vi "UHR-Fleezers Control (host) - 12.7c.vi"() -> ()   [LabVIEW 2012] (continued)
          tunnel: w2948 -> [w2975]
          tunnel: w2947 -> [w2974]
          frame #0 {
            n2017 = call "Read Stage Position.vi"("error in"=w2965, "VISA resource name in"=w2957) -> ("Current Position"=w2955:cluster{dbl, dbl, dbl}, "error out"=w2958:errorcluster, "VISA resource name out"=w2956:refnum<visa-resource-name>)  [unwired: 1 out]
            "Current Position" <- w2955
            n2018 = local write "Stage Control Serial Error"(w2958) -> ()
            n2019 = Unbundle(w2955) -> (w2962:dbl, w2964:dbl, w2960:dbl)
            n2020 = Add(x=w2964, y="Y change (mm)") -> (x+y=w2961:dbl)
            n2021 = Bundle(w2962, w2961, w2960) -> (w2959:cluster{dbl, dbl, dbl})  [unwired: 1 in]
          }
          frame #1 {
            # "move to new position and start saving"
            n2022 = local write "Stage Moving"(TRUE ("Stage Moving")) -> ()
            n2023 = local write "Start Saving"(TRUE ("Start Saving")) -> ()
            n2024 = call "Set Stage Position.vi"("Position"=w2972, "error in"=w2971, "VISA resource name in"=w2970) -> ("error out"=w2968:errorcluster, "VISA resource name out"=w2969:refnum<visa-resource-name>)  [unwired: 1 out]
          }
          frame #2 {
            # "go back to start"
            n2025 = call "Set Stage Position.vi"("Position"=w2974, "error in"=w2975, "VISA resource name in"=w2976) -> ()  [unwired: 3 out]
          }
          frame #3 {
            # "stop saving"
            n2026 = local write "Stop Saving"(TRUE ("Stop Saving")) -> ()
            n2027 = local write "Stage Moving"(FALSE ("Stage Moving")) -> ()
          }
        }
      }
      event "Move to Position 1", "Move to Position 2", "Move to Position 3", "Move to Position 4", "Move to Position 5", "Lower Ch. Cap.": Value Change {
        n2028 = event-data() -> ()  [unwired: 1 in, 5 out]
        n2029 = Or(x="Move to Position 5", y="Lower Ch. Cap.") -> (x .or. y?=w2982:bool)
        n2030 = Build Array("Move to Position 1", "Move to Position 2", "Move to Position 3", "Move to Position 4", w2982) -> (w2985:bool[])
        n2031 = Boolean Array To Number(Boolean array=w2985) -> (number=w2984:u32)
        n2032 = Logarithm Base 2(1:w2984) -> (0:w2983:dbl)
        n2033 = flat-sequence {
          tunnel: w2983 -> [w2994]
          tunnel: w2980 -> [w2992]
          tunnel: w2979 -> [w2991]
          frame #0 {
            n2034 = local read "Saved Stage Positions"() -> (w3002:dbl[][])
            n2035 = Array Subset(array=w3002, index (row)=w2994, length (row)=1 ("length"), index (col)=1 ("index"), length (col)=3 ("length")) -> (w2999:dbl[][])
            n2036 = Reshape Array(w2999, 3 ("dimension size")) -> (w2997:dbl[])
            n2037 = Array To Cluster(array=w2997) -> (cluster=w2996:cluster{"[0]":dbl, "[1]":dbl, "[2]":dbl})
            n2038 = call "Set Stage Position.vi"("Position"=w2996, "error in"=w2991, "VISA resource name in"=w2992) -> ("error out"=w2995:errorcluster)  [unwired: 2 out]
            n2039 = local write "Stage Moving"(TRUE ("Stage Moving")) -> ()
            n2040 = local write "Stage Control Serial Error"(w2995) -> ()
          }
          frame #1 {
            n2041 = local write "Stage Moving"(FALSE ("Stage Moving")) -> ()
            n2042 = call <vilib>:"Beep.vi"() -> ()  [unwired: 3 in, 9 out]
          }
        }
      }
      event "Got ADig bead": Value Change {
        n2043 = event-data() -> ()  [unwired: 1 in, 5 out]
        n2044 = flat-sequence {
          frame #0 {
            n2045 = local read "Cap 1 Samp Flow ON"() -> (w3006:bool)
            n2046 = case shown="True" w3006 {
              frame False {
              }
              frame True {
                n2047 = property on="Sample Channel\nFlow" class="Bool (strict)"("Val(Sgnl)"=TRUE ("Value (Signaling)")) -> ()  [unwired: 2 in, 2 out]
              }
            }
          }
          frame #1 {
            n2048 = property on="Inject Pump 3" class="Bool (strict)"("Val(Sgnl)"=FALSE ("Value (Signaling)")) -> ()  [unwired: 2 in, 2 out]
          }
          frame #2 {
            n2049 = property on="Move Cap. 1 (DNA Bottom)" class="Bool (strict)"("Val(Sgnl)"=TRUE ("Value (Signaling)")) -> ()  [unwired: 2 in, 2 out]
          }
        }
      }
      event "Force FB Data\nScript": Value Change {
        n2050 = event-data() -> ()  [unwired: 1 in, 5 out]
        n2051 = flat-sequence {
          tunnel: w3015 -> [w3019]
          tunnel: w3016 -> [w3020]
          tunnel: [w3020] -> w3011
          tunnel: [w3019] -> w3010
          tunnel: w3011 -> [w3023]
          tunnel: w3010 -> [w3022]
          tunnel: ["Trap Trig Fl."] -> w3012
          tunnel: [w3048] -> w3013
          tunnel: w3012 -> [w3048]
          tunnel: [w3052] -> w3014
          tunnel: w3013 -> [w3052]
          tunnel: w3014 -> [w3054]
          frame #0 {
            n2052 = property on="Trap Delta (MHz)" class="DigNum (strict)"("Val(Sgnl)"="Trap Delta Before Moving") -> ()  [unwired: 2 in, 2 out]
          }
          frame #1 {
            n2053 = local read "Saved Stage Positions"() -> (w3025:dbl[][])
            n2054 = local write "FB Trap Pos Offset"(0.0 ("FB Trap Pos Offset")) -> ()
            n2055 = property on="Trap Pos. FB Offset Factor" class="DigNum (strict)"("Val(Sgnl)"=i64 0 ("Value (Signaling)")) -> ()  [unwired: 2 in, 2 out]
            n2056 = local write "Stage Moving"(TRUE ("Stage Moving")) -> ()
            n2057 = call "move to saved stage position.vi"("error in"=w3022, "Stage VISA resource name in"=w3023, "Position"="Stage Position To Establish FB", "Saved Stage Positions"=w3025) -> ("error out"=w3021:errorcluster)  [unwired: 1 out]
            n2058 = local write "Stage Control Serial Error"(w3021) -> ()
          }
          frame #2 {
            n2059 = call <vilib>:"Beep.vi"() -> ()  [unwired: 3 in, 9 out]
            n2060 = Multiply(x="Wait (s)", y=u32 1000 ("milliseconds to wait")) -> (x*y=w3032:u32)
            n2061 = property on="Trap Delta (MHz)" class="DigNum (strict)"("Val(Sgnl)"="Starting \nTrap Delta (MHz)") -> ()  [unwired: 2 in, 2 out]
            n2062 = local write "Stage Moving"(FALSE ("Stage Moving")) -> ()
            n2063 = Wait (ms)(milliseconds to wait=w3032) -> ()  [unwired: 1 out]
            n2064 = property on="Tab Control 2" class="TabCtl (strict)"("Val(Sgnl)"=T6."Feedback on Trap Position" ("Value (Signaling)")) -> ()  [unwired: 2 in, 2 out]
            n2065 = property on="Tab Control" class="TabCtl (strict)"("Val(Sgnl)"=T34."Trap Control (RF)" ("Value (Signaling)")) -> ()  [unwired: 2 in, 2 out]
          }
          frame #3 {
            n2066 = property on="Set Reading to\nSetpoint" class="Bool (strict)"("Val(Sgnl)"=TRUE ("Value (Signaling)")) -> ()  [unwired: 2 in, 2 out]
            n2067 = Wait (ms)(milliseconds to wait=u32 500) -> ()  [unwired: 1 out]
          }
          frame #4 {
            n2068 = property on="Trap Pos. FB ON" class="Bool (strict)"("Val(Sgnl)"=TRUE ("Value (Signaling)")) -> ()  [unwired: 2 in, 2 out]
            n2069 = Wait (ms)(milliseconds to wait=u32 250) -> ()  [unwired: 1 out]
          }
          frame #5 {
            n2070 = case shown="False" "Trap Trig Fl." {
              frame False {
                n2071 = case shown="True" "Green ON after FB ON?" {
                  selector: "Green ON after FB ON?" -> [_ w3047]
                  frame False {
                  }
                  frame True {
                    n2072 = property on="Green Laser ON" class="Bool (strict)"("Val(Sgnl)"=w3047) -> ()  [unwired: 2 in, 2 out]
                  }
                }
              }
              frame True {
              }
            }
            n2073 = case shown="True" "Remove Action Offset" {
              tunnel: TRUE ("Value (Signaling)") -> [w3044 w3045]
              frame False {
                n2074 = property on="Remove Unwinding Offset" class="Bool (strict)"("Val(Sgnl)"=w3044) -> ()  [unwired: 2 in, 2 out]
              }
              frame True {
                n2075 = property on="Remove Action Offset" class="Bool (strict)"("Val(Sgnl)"=w3045) -> ()  [unwired: 2 in, 2 out]
              }
            }
            n2076 = Wait (ms)(milliseconds to wait=u32 250) -> ()  [unwired: 1 out]
          }
          frame #6 {
            n2077 = property on="Start Saving" class="Bool (strict)"("Val(Sgnl)"=TRUE ("Value (Signaling)")) -> ()  [unwired: 2 in, 2 out]
            n2078 = Wait (ms)(milliseconds to wait=u32 5000) -> ()  [unwired: 1 out]
          }
          frame #7 {
            w3051 = TRUE ("Value (Signaling)")
            n2079 = property on="Rem fb disp offset" class="Bool (strict)"("Val(Sgnl)"=w3051) -> ()  [unwired: 2 in, 2 out]
            n2080 = property on="Remove Offset" class="Bool (strict)"("Val(Sgnl)"=w3051) -> ()  [unwired: 2 in, 2 out]
            n2081 = Wait (ms)(milliseconds to wait=u32 100) -> ()  [unwired: 1 out]
          }
          frame #8 {
            n2082 = case shown="True" w3054 {
              frame False {
              }
              frame True {
                n2083 = local write "Trap Trig. Fl."(TRUE ("Value (Signaling)")) -> ()
              }
            }
          }
          frame #9 {
            n2084 = case shown="True" "Start dipping after?" {
              frame False {
              }
              frame True {
                n2085 = flat-sequence {
                  frame #0 {
                    n2086 = Multiply(x="Delay before dipping (s)", y=1000.0) -> (x*y=w3058:dbl)
                    n2087 = Wait (ms)(milliseconds to wait=w3058) -> ()  [unwired: 1 out]
                  }
                  frame #1 {
                    n2088 = property on="Dip for Protein" class="Bool (strict)"("Val(Sgnl)"=TRUE ("Value (Signaling)")) -> ()  [unwired: 2 in, 2 out]
                    n2089 = local write "Scripts"(T1."Dipping" ("Scripts")) -> ()
                  }
                }
              }
            }
          }
        }
      }
      event "Fixed Traps Data\nScript": Value Change {
        n2090 = event-data() -> ()  [unwired: 1 in, 5 out]
        n2091 = flat-sequence {
          frame #0 {
            n2092 = case shown="True" "Green ON" {
              frame False {
              }
              frame True {
                n2093 = property on="Green Laser ON" class="Bool (strict)"("Val(Sgnl)"=TRUE) -> ()  [unwired: 2 in, 2 out]
              }
            }
            n2094 = local write "Offset (nm)"(0.0 ("Offset (nm)")) -> ()
            n2095 = property on="Sample Channel\nFlow" class="Bool (strict)"("Val(Sgnl)"=FALSE ("Value (Signaling)")) -> ()  [unwired: 2 in, 2 out]
            n2096 = property on="Trap Delta (MHz)" class="DigNum (strict)"("Val(Sgnl)"="Fixed Traps Trap Delta (MHz)") -> ()  [unwired: 2 in, 2 out]
          }
          frame #1 {
            n2097 = Wait (ms)(milliseconds to wait=u32 1000) -> ()  [unwired: 1 out]
          }
          frame #2 {
            n2098 = local write "Start Saving"(TRUE ("Start Saving")) -> ()
          }
          frame #3 {
            n2099 = local read "Bead Sep. Int. Time (s)"() -> (w3069:dbl)
            n2100 = Multiply(x=w3069, y=1000.0) -> (x*y=w3071:dbl)
            n2101 = Wait (ms)(milliseconds to wait=w3071) -> ()  [unwired: 1 out]
          }
          frame #4 {
            n2102 = property on="Remove Offset" class="Bool (strict)"("Val(Sgnl)"=TRUE ("Value (Signaling)")) -> ()  [unwired: 2 in, 2 out]
          }
          frame #5 {
            n2103 = property on="Dip for Protein" class="Bool (strict)"("Val(Sgnl)"="Start dipping after?") -> ()  [unwired: 2 in, 2 out]
          }
        }
      }
      event "Got DNA bead": Value Change {
        n2104 = event-data() -> ()  [unwired: 1 in, 5 out]
        n2105 = flat-sequence {
          frame #0 {
            n2106 = local read "Daq spot flow on"() -> (w3076:bool)
            n2107 = case shown="True" w3076 {
              frame False {
              }
              frame True {
                n2108 = property on="Sample Channel\nFlow" class="Bool (strict)"("Val(Sgnl)"=TRUE ("Value (Signaling)")) -> ()  [unwired: 2 in, 2 out]
              }
            }
            n2109 = property on="Got DNA bead" class="Bool"("Key Focus"=FALSE) -> ()  [unwired: 2 in, 2 out]
          }
          frame #1 {
            n2110 = property on="Inject Pump 1" class="Bool (strict)"("Val(Sgnl)"=FALSE ("Value (Signaling)")) -> ()  [unwired: 2 in, 2 out]
          }
          frame #2 {
            n2111 = property on="Cal/Data Acq. Spot" class="Bool (strict)"("Val(Sgnl)"=TRUE ("Value (Signaling)")) -> ()  [unwired: 2 in, 2 out]
          }
        }
      }
      event "Take Stepping Data": Value Change {
        n2112 = event-data() -> ()  [unwired: 1 in, 5 out]
        n2113 = local read "Save ave N"() -> (w3088:dbl)
        n2114 = flat-sequence {
          tunnel: w3088 -> [w3090]
          tunnel: [w3090] -> w3083
          tunnel: [w3092] -> w3084
          tunnel: w3083 -> [w3092]
          tunnel: [w3094] -> w3085
          tunnel: w3084 -> [w3094]
          tunnel: [w3097] -> w3086
          tunnel: w3085 -> [w3097]
          tunnel: [w3099] -> w3087
          tunnel: w3086 -> [w3099]
          tunnel: [w3101] -> w3081
          tunnel: w3087 -> [w3101]
          tunnel: w3081 -> [w3104]
          tunnel: [w3104] -> w3080
          tunnel: w3080 -> [w3105]
          tunnel: [w3105] -> w3082
          tunnel: w3082 -> [w3111]
          frame #0 {
            n2115 = property on="Save ave N" class="DigNum (strict)"("Val(Sgnl)"="Save ave factor") -> ()  [unwired: 2 in, 2 out]
          }
          frame #1 {
            n2116 = Wait (ms)(milliseconds to wait=u32 100) -> ()  [unwired: 1 out]
          }
          frame #2 {
            n2117 = local read "Offset 2 Start (MHz)"() -> (w3096:dbl)
            n2118 = property on="Saved AOD Raster Scan Parameter Sets" class="Arr (strict)"("Index Values"=u32[] [2]) -> ()  [unwired: 2 in, 2 out]
            n2119 = property on="Trap Delta (MHz)" class="DigNum (strict)"("Val(Sgnl)"=w3096) -> ()  [unwired: 2 in, 2 out]
          }
          frame #3 {
            n2120 = property on="Load parameters" class="Bool (strict)"("Val(Sgnl)"=TRUE ("Value (Signaling)")) -> ()  [unwired: 2 in, 2 out]
          }
          frame #4 {
            n2121 = Wait (ms)(milliseconds to wait=u32 100) -> ()  [unwired: 1 out]
          }
          frame #5 {
            n2122 = property on="Trap Raster Scan" class="Bool (strict)"("Val(Sgnl)"=TRUE ("Value (Signaling)")) -> ()  [unwired: 2 in, 2 out]
          }
          frame #6 {
            n2123 = Wait (ms)(milliseconds to wait=u32 1000) -> ()  [unwired: 1 out]
          }
          frame #7 {
            n2124 = while {
              stop <- w3108 stop-if-true
              n2125 = local read "Raster Scanning..."() -> (w3110:bool)
              n2126 = local read "Saving..."() -> (w3109:bool)
              n2127 = Not(x=w3109) -> (.not. x?=w3106:bool)
              n2128 = Not(x=w3110) -> (.not. x?=w3107:bool)
              n2129 = And(x=w3107, y=w3106) -> (x .and. y?=w3108:bool)
            }
          }
          frame #8 {
            n2130 = property on="Save ave N" class="DigNum (strict)"("Val(Sgnl)"=w3111) -> ()  [unwired: 2 in, 2 out]
          }
        }
      }
      event "Step Size (nm)": Value Change {
        n2131 = event-data() -> ()  [unwired: 1 in, 5 out]
        n2132 = flat-sequence {
          frame #0 {
            n2133 = property on="Saved AOD Raster Scan Parameter Sets" class="Arr (strict)"("Index Values"=u32[] [1]) -> ()  [unwired: 2 in, 2 out]
          }
          frame #1 {
            n2134 = Multiply(x="N Steps", y="Step Size (nm)") -> (x*y=w3113:dbl)
            n2135 = property on="Scan Speed AOD (nm/s) 2" class="DigNum (strict)"("Value"="Step Size (nm)") -> ()  [unwired: 2 in, 2 out]
            n2136 = property on="Step Size AOD (nm) 2" class="DigNum (strict)"("Value"="Step Size (nm)") -> ()  [unwired: 2 in, 2 out]
            n2137 = property on="Scan Range AOD (nm) 2" class="DigNum (strict)"("Value"=w3113) -> ()  [unwired: 2 in, 2 out]
          }
        }
      }
      event "Take Detection Laser\nImage": Value Change {
        n2138 = event-data() -> ()  [unwired: 1 in, 5 out]
        n2139 = flat-sequence {
          tunnel: [w3141] -> w3131
          tunnel: [w3140] -> w3124
          tunnel: [w3139] -> w3116
          tunnel: [w3144] -> w3132
          tunnel: w3131 -> [w3144]
          tunnel: [w3143] -> w3125
          tunnel: w3124 -> [w3143]
          tunnel: [w3142] -> w3117
          tunnel: w3116 -> [w3142]
          tunnel: [w3148] -> w3133
          tunnel: w3132 -> [w3148]
          tunnel: [w3147] -> w3126
          tunnel: w3125 -> [w3147]
          tunnel: [w3146] -> w3118
          tunnel: w3117 -> [w3146]
          tunnel: [w3154] -> w3134
          tunnel: w3133 -> [w3154]
          tunnel: [w3153] -> w3127
          tunnel: w3126 -> [w3153]
          tunnel: [w3152] -> w3119
          tunnel: w3118 -> [w3152]
          tunnel: [w3158] -> w3135
          tunnel: w3134 -> [w3158]
          tunnel: [w3157] -> w3128
          tunnel: w3127 -> [w3157]
          tunnel: [w3156] -> w3120
          tunnel: w3119 -> [w3156]
          tunnel: [w3162] -> w3136
          tunnel: w3135 -> [w3162]
          tunnel: [w3161] -> w3129
          tunnel: w3128 -> [w3161]
          tunnel: [w3160] -> w3121
          tunnel: w3120 -> [w3160]
          tunnel: [w3166] -> w3137
          tunnel: w3136 -> [w3166]
          tunnel: [w3165] -> w3130
          tunnel: w3129 -> [w3165]
          tunnel: [w3164] -> w3122
          tunnel: w3121 -> [w3164]
          tunnel: w3137 -> [w3172]
          tunnel: w3130 -> [w3171]
          tunnel: [w3169] -> w3123
          tunnel: w3122 -> [w3169]
          tunnel: w3123 -> [w3173]
          frame #0 {
            n2140 = local read "Laser interlacing mode"() -> (w3140:enum32{"Laser ON", "Laser OFF", "Interlace"})
            n2141 = local read "Green FB On/Off"() -> (w3139:bool)
            n2142 = local read "Green Laser ON"() -> (w3141:bool)
          }
          frame #1 {
            n2143 = property on="Green FB On/Off" class="Bool (strict)"("Val(Sgnl)"=FALSE ("Value (Signaling)")) -> ()  [unwired: 2 in, 2 out]
          }
          frame #2 {
            n2144 = property on="Green Laser ON" class="Bool (strict)"("Val(Sgnl)"=TRUE ("Value (Signaling)")) -> ()  [unwired: 2 in, 2 out]
            n2145 = property on="Flip Green Filter" class="Bool (strict)"("Val(Sgnl)"=TRUE ("Value (Signaling)")) -> ()  [unwired: 2 in, 2 out]
            n2146 = property on="Laser interlacing mode" class="RadioBtnsControl (strict)"("Val(Sgnl)"=enum32{"Laser ON", "Laser OFF", "Interlace"}."Laser ON" ("Value (Signaling)")) -> ()  [unwired: 2 in, 2 out]
          }
          frame #3 {
            n2147 = Wait (ms)(milliseconds to wait=u32 500) -> ()  [unwired: 1 out]
          }
          frame #4 {
            n2148 = property on="Confocal Image" class="Bool (strict)"("Val(Sgnl)"=TRUE ("Value (Signaling)")) -> ()  [unwired: 2 in, 2 out]
          }
          frame #5 {
            n2149 = Wait (ms)(milliseconds to wait=u32 2000) -> ()  [unwired: 1 out]
          }
          frame #6 {
            n2150 = while {
              stop <- w3167 stop-if-true
              n2151 = local read "Saving..."() -> (w3168:bool)
              n2152 = Not(x=w3168) -> (.not. x?=w3167:bool)
            }
          }
          frame #7 {
            n2153 = property on="Flip Green Filter" class="Bool (strict)"("Val(Sgnl)"=TRUE ("Value (Signaling)")) -> ()  [unwired: 2 in, 2 out]
            n2154 = property on="Green Laser ON" class="Bool (strict)"("Val(Sgnl)"=w3172) -> ()  [unwired: 2 in, 2 out]
            n2155 = property on="Laser interlacing mode" class="RadioBtnsControl (strict)"("Val(Sgnl)"=w3171) -> ()  [unwired: 2 in, 2 out]
          }
          frame #8 {
            n2156 = property on="Green FB On/Off" class="Bool (strict)"("Val(Sgnl)"=w3173) -> ()  [unwired: 2 in, 2 out]
          }
        }
      }
      event "Move in a Circle": Value Change {
        w3184 = dbl[] []
        # "converting distance (d) to angle (a)\na=arcsin(d/2r)"
        # "radius"
        # "radius"
        # "T1 Y"
        # "T1 X"
        n2157 = event-data() -> ()  [unwired: 1 in, 5 out]
        n2158 = local read "BD 1 Frequency 1 (MHz)"() -> (w3181:dbl)
        n2159 = local read "BD 2 Frequency 1 (MHz)"() -> (w3180:dbl)
        n2160 = local read "BD 1 Frequency 2 (MHz)"() -> (w3179:dbl)
        n2161 = local read "BD 2 Frequency 2 (MHz)"() -> (w3178:dbl)
        n2162 = Subtract(x=w3180, y="Center Y Frequency (MHz)") -> (x-y=w3186:dbl)
        n2163 = Absolute Value(x=w3186) -> (abs(x)=w3176:dbl)
        n2164 = flat-sequence {
          tunnel: w3176 -> [w3189]
          tunnel: [w3189] -> w3175
          frame #0 {
            n2165 = local write "Radius (MHz)"(w3189) -> ()
          }
        }
        n2166 = node-c288("Time step (ms)") -> (w3188:T23)  [unwired: 3 in]
        n2167 = timed-loop {
          timing: w3188 -> [_]
          timing-out: [_] -> w3187
          tunnel: w3181 -> [w3246]
          tunnel: w3180 -> [_]
          tunnel: w3179 -> [w3250]
          tunnel: w3178 -> [_]
          tunnel: "Center Y Frequency (MHz)" -> [w3227]
          shift-right: [w3237] -> _
          shift-left: w3184 -> [w3239]
          shift-right: [w3236] -> _
          shift-left: w3184 -> [w3238]
          shift-right: [w3234] -> _
          shift-left: w3184 -> [w3233]
          shift-right: [w3232] -> _
          shift-left: w3184 -> [w3231]
          tunnel: "Move in a Circle" -> [_]
          tunnel: ["Back to start on finish?"] -> w3177
          tunnel: w3175 -> [_]
          tunnel: w3174 -> [w3204]
          i -> [w3226]
          stop <- w3244 stop-if-true
          # "Trap 2"
          # "Trap 1"
          # "ignore if N = 0"
          # "r"
          # "r"
          # "r"
          # "r"
          # "\"omega*t\""
          # "Trap 2"
          # "Trap separation (radians)"
          # "Trap 1"
          # "Offset (starts\n at bottom of\n the circle)"
          # "\"t\""
          # "omega"
          n2168 = node-c288() -> (w3259:i64)  [unwired: 1 in]
          n2169 = Divide(x=w3259, y=1000) -> (x/y=w3258:dbl)
          n2170 = Divide(x="2D Motion Trap Separation (MHz)", y="Radius (MHz)") -> (x/y=w3214:dbl)
          n2171 = Multiply(x=w3258, y=w3226) -> (x*y=w3218:dbl)
          n2172 = Inverse Sine(1:w3214) -> ()  [unwired: 1 out]
          n2173 = Multiply(x=w3218, y=-1.0) -> (x*y=w3219:dbl)
          n2174 = Multiply(x=6.283185307179586, y="2D Motion Frequency (Hz)") -> (x*y=w3229:dbl)
          n2175 = Select(t=w3218, s="Counterclockwise/Clockwise", f=w3219) -> (s? t:f=w3217:dbl)
          n2176 = Multiply(x=w3229, y=w3217) -> (x*y=w3240:dbl)
          n2177 = Divide(x="Trap 2 phase shift (deg)", y=6.283185307179586) -> (x/y=w3199:dbl)
          n2178 = Add(x=w3240, y=w3199) -> (x+y=w3211:dbl)
          n2179 = Add(x=w3240, y=1.5707963267948966) -> (x+y=w3256:dbl)
          n2180 = Add(x=w3211, y=1.5707963267948966) -> (x+y=w3241:dbl)
          n2181 = Cosine(x=w3256) -> (cos(x)=w3255:dbl)
          n2182 = Sine(x=w3256) -> (sin(x)=w3254:dbl)
          n2183 = Multiply(x=w3255, y="Radius (MHz)") -> (x*y=w3248:dbl)
          n2184 = Cosine(x=w3241) -> (cos(x)=w3253:dbl)
          n2185 = Sine(x=w3241) -> (sin(x)=w3252:dbl)
          n2186 = Multiply(x=w3254, y="Radius (MHz)") -> (x*y=w3247:dbl)
          n2187 = Multiply(x=w3253, y="Radius (MHz)") -> (x*y=w3251:dbl)
          n2188 = Multiply(x=w3252, y="Radius (MHz)") -> (x*y=w3249:dbl)
          n2189 = Add(x=w3248, y=w3246) -> (x+y=w3210:dbl)
          n2190 = Add(x=w3247, y=w3227) -> (x+y=w3208:dbl)
          n2191 = Greater Or Equal?(x=w3226, y="N steps then stop") -> (x >= y?=w3225:bool)
          n2192 = Add(x=w3251, y=w3250) -> (x+y=w3209:dbl)
          n2193 = Add(x=w3249, y=w3227) -> (x+y=w3207:dbl)
          n2194 = Not Equal To 0?(x="N steps then stop") -> (x != 0?=w3221:bool)
          n2195 = And(x=w3225, y=w3221) -> (x .and. y?=w3222:bool)
          n2196 = local read "Stop All"() -> (w3243:bool)
          n2197 = local write "BD 1 Frequency 1 (MHz)"(w3210) -> ()
          n2198 = local write "BD 2 Frequency 1 (MHz)"(w3208) -> ()
          n2199 = local write "BD 1 Frequency 2 (MHz)"(w3209) -> ()
          n2200 = local write "BD 2 Frequency 2 (MHz)"(w3207) -> ()
          n2201 = Compound Arithmetic op=OR(w3243, "Stop Moving", w3222) -> (w3244:bool)
          n2202 = local read "BD 1 Frequency 3 (MHz)"() -> (w3206:dbl)
          n2203 = local read "BD 2 Frequency 3 (MHz)"() -> (w3205:dbl)
          n2204 = local read "Y RF Frequency Limits (MHz)"() -> (w3202:T16)
          n2205 = local read "X RF Frequency Limits (MHz)"() -> (w3203:T16)
          n2206 = call "set RF board frequency - interlace.vi"("Board 2 Frequency Limits"=w3202, "Board 1 Frequency Limits"=w3203, "FPGA VI Reference In"=w3204, "Board 2 Frequency 3 (MHz)"=w3205, "Board 1 Frequency 3 (MHz)"=w3206, "Board 2 Frequency 2 (MHz)"=w3207, "Board 2 Frequency 1 (MHz)"=w3208, "Board 1 Frequency 2 (MHz)"=w3209, "Board 1 Frequency 1  (MHz)"=w3210) -> ()  [unwired: 1 in, 2 out]
          n2207 = Build Array (concatenate)(w3239, w3210) -> (w3237:dbl[])
          n2208 = Build Array (concatenate)(w3238, w3208) -> (w3236:dbl[])
          n2209 = Build Array (concatenate)(w3233, w3209) -> (w3234:dbl[])
          n2210 = Build Array (concatenate)(w3231, w3207) -> (w3232:dbl[])
          n2211 = Bundle(w3237, w3236) -> (→"Trap 1 trajectory":cluster{dbl[], dbl[]})  [unwired: 1 in]
          n2212 = Bundle(w3234, w3232) -> (→"Trap 2 trajectory":cluster{dbl[], dbl[]})  [unwired: 1 in]
          n2213 = node-c288() -> ()  [unwired: 1 in, 1 out]
        }
        n2214 = node-c288(w3187) -> ()  [unwired: 1 out]
        n2215 = case shown="True" w3177 {
          tunnel: w3181 -> [_ w3193]
          tunnel: w3180 -> [_ w3192]
          tunnel: w3179 -> [_ w3191]
          tunnel: w3178 -> [_ w3190]
          frame False {
          }
          frame True {
            n2216 = flat-sequence {
              tunnel: w3193 -> [w3197]
              tunnel: w3192 -> [w3196]
              tunnel: w3191 -> [w3195]
              tunnel: w3190 -> [w3194]
              frame #0 {
                n2217 = local write "BD 1 Frequency 1 (MHz)"(w3197) -> ()
                n2218 = local write "BD 2 Frequency 1 (MHz)"(w3196) -> ()
                n2219 = local write "BD 1 Frequency 2 (MHz)"(w3195) -> ()
                n2220 = local write "BD 2 Frequency 2 (MHz)"(w3194) -> ()
              }
              frame #1 {
                n2221 = property on="Update all trap values" class="Bool (strict)"("Val(Sgnl)"=TRUE ("Value (Signaling)")) -> ()  [unwired: 2 in, 2 out]
              }
            }
          }
        }
      }
      event "Stop All": Value Change {
        # "Stopping blue laser before shutting off program"
        n2222 = event-data() -> ()  [unwired: 1 in, 5 out]
        n2223 = local read "Delay (ms)"() -> (w3270:i32)
        n2224 = call "serial write macro.vi"("String"="l0", "Delay (ms)"=w3270, "VISA resource name"=w3273) -> ("read buffer"=w3268:string, "error out"=w3269:errorcluster, "VISA resource name out"=w3272:refnum<visa-resource-name>)
        n2225 = local write "read blue buffer"(w3268) -> ()
        n2226 = local write "Blue Error Out"(w3269) -> ()
        n2227 = VISA Close(VISA resource name=w3272) -> ()  [unwired: 1 in, 1 out]
        n2228 = local read "Stop All"() -> (w3274:bool)
      }
    }
    n2229 = node-c288() -> ()  [unwired: 1 in, 1 out]
  }
  n2230 = flat-sequence "Video" {
    tunnel: [w3284] -> w121
    tunnel: w121 -> [w3324]
    frame #0 {
      n2231 = while {
        stop <- w3276 continue-if-true
        n2232 = call "Close Video Capture.vi"() -> ("error code OUT"=w3278:i32)
        n2233 = Equal?(x=w3278, y=0) -> (x = y?=w3276:bool)
      }
      n2234 = local write "Stop All"(FALSE ("Stop All")) -> ()
    }
    frame #1 {
      n2235 = call "DMR_Init.vi"() -> ()  [unwired: 3 out]
    }
    frame #2 {
      w3279 = "DE245428202"  # MSU fleezers card #
      (unwired) "DE019116701"  # Illinois fleezers card #
      # "Setting the destination format to Mono8 makes sure that the image can be displayed in the intensity plot."
      n2236 = call "DMR_GetDevice.vi"("search string IN"=w3279) -> ("device handle OUT"=w3302:i32)  [unwired: 4 in, 2 out]
      n2237 = call "DMR_OpenDevice.vi"("device handle IN"=w3302) -> ("driver handle OUT"=w3285:i32)  [unwired: 4 out]
      n2238 = call "DMR_FindList.vi"("flags IN"=u32 0 ("flags"), "list name IN"="" ("String"), "list type IN"=T35."camera descriptions", "driver handle IN"=w3285) -> ("list handle OUT"=w3288:i32)  [unwired: 2 out]
      n2239 = call "DMR_FindList.vi"("flags IN"=u32 0 ("flags"), "list name IN"="Base", "list type IN"=T35."setting", "driver handle IN"=w3285) -> ("list handle OUT"=w3286:i32)  [unwired: 2 out]
      n2240 = call "OBJ_GetHandle.vi"("object name IN"="VideoStandard", "list handle IN"=w3288) -> ("object handle OUT"=w3282:i32)  [unwired: 3 out]
      n2241 = call "OBJ_GetHandle.vi"("object name IN"="PixelFormat", "list handle IN"=w3286) -> ("object handle OUT"=w3296:i32)  [unwired: 3 out]
      n2242 = call "OBJ_SetS.vi"("value index IN"=0, "value IN"="NTSC M", "object handle IN"=w3282) -> ()  [unwired: 2 out]
      n2243 = call "OBJ_SetS.vi"("value index IN"=0, "value IN"="Mono8" ("value"), "object handle IN"=w3296) -> ()  [unwired: 2 out]
      n2244 = call "OBJ_GetHandle.vi"("object name IN"="VideoChannel", "list handle IN"=w3286) -> ("object handle OUT"=w3292:i32)  [unwired: 3 out]
      n2245 = while {
        tunnel: [w3306] -> w3284
        tunnel: w3285 -> [w3303]
        stop <- w3304 continue-if-true
        n2246 = call "DMR_ImageRequestSingle.vi"("request control IN"=0, "driver handle IN"=w3303) -> ("error code OUT"=w3305:i32, "driver handle OUT"=w3306:i32)  [unwired: 2 out]
        n2247 = Equal To 0?(x=w3305) -> (x = 0?=w3304:bool)
      }
      n2248 = call "OBJ_SetI.vi"("value index IN"=0, "value IN"=3 ("Video channel"), "object handle IN"=w3292) -> ()  [unwired: 2 out]
    }
    frame #3 {
      w3312 = T18 0 items=["Grayscale (U8)", "Grayscale (I16)", "Grayscale (SGL)", "Complex (CSG)", "RGB (U32)", "HSL (U32)", "RGB (U64)"] ("Image Type")
      w3320 = T18 0 items=["Grayscale (U8)", "Grayscale (I16)", "Grayscale (SGL)", "Complex (CSG)", "RGB (U32)", "HSL (U32)", "RGB (U64)"] ("Image Type")
      n2249 = for "Create Greyscale map" {
        N: 256 -> [_]
        tunnel: [w3326] -> w3309 mode=indexing
        workers-P: _ -> [_]
        i -> [w3329]
        n2250 = To Unsigned Byte Integer(number=w3329) -> (unsigned 8bit integer=w3325:u8)
        n2251 = Join Numbers(hi=w3325, lo=w3325) -> ((hi.lo)=w3328:u16)
        n2252 = Join Numbers(hi=w3325, lo=w3325) -> ((hi.lo)=w3327:u16)
        n2253 = Join Numbers(hi=w3328, lo=w3327) -> ((hi.lo)=w3326:u32)
      }
      n2254 = call "IMAQ Create"("Image Name"="Scaled video", "Image Type"=w3312) -> ("New Image"=w3311:T2)  [unwired: 2 in, 2 out]
      n2255 = call "IMAQ Create"("Image Name"="Main video", "Image Type"=w3320) -> ("New Image"=w3321:T2)  [unwired: 2 in, 2 out]
      n2256 = node-c288(0 ("Processor")) -> (w3319:T23)  [unwired: 3 out]
      n2257 = Initialize Array(u32 0 ("Window Number (0...15)"), 480 ("dimension size"), 640 ("dimension size")) -> (w3314:u32[][])
      n2258 = timed-loop {
        tunnel: w3324 -> [w3346]
        tunnel: [w3345] -> w3323
        tunnel: w3321 -> [w3344]
        timing: w3319 -> [_]
        timing-out: [_] -> w3318
        tunnel: w3314 -> [w3333]
        tunnel: w3311 -> [w3331]
        tunnel: w3309 -> [w3330]
        stop <- w3332 stop-if-true
        # "This block performs the \nactual image capture."
        n2259 = node-c288() -> ()  [unwired: 2 out]
        n2260 = local read "Stop All"() -> (w3332:bool)
        n2261 = Reciprocal(x="Video Capture Rate (Hz)") -> (1/x=w3336:dbl)
        n2262 = Multiply(x=w3336, y=1000.0) -> (x*y=w3334:dbl)
        n2263 = call "DMR_ImageRequestWaitFor.vi"("queue number IN"=0, "timeout(ms) IN"=500, "driver handle IN"=w3346) -> ("error code OUT"=w3350:i32, "request number OUT"=w3347:i32, "driver handle OUT"=w3348:i32)
        n2264 = feedback #1(T36 refnum ("Avi Refnum")) -> (w3338:T36)
        n2265 = case shown="True" "New Video File" {
          tunnel: [T36 refnum ("Avi Refnum") w3367] -> w3340
          tunnel: [FALSE TRUE] -> w3341
          tunnel: w3338 -> [_ w3363]
          frame False {
          }
          frame True {
            n2266 = call "Create new save file.vi"("Ext"=".avi" ("string"), "Index In"="Video Index") -> ("Path Out"=w3359:path, "Index Out"=w3360:dbl)  [unwired: 1 in]
            "Path Out" <- w3359
            n2267 = Not Equal?(x=w3363, y=T36 refnum ("Avi Refnum")) -> (x != y?=w3364:bool)
            n2268 = Increment(x=w3360) -> (x+1=w3369:dbl)
            n2269 = case shown="True" w3364 {
              tunnel: w3363 -> [_ w3370]
              frame False {
              }
              frame True {
                n2270 = call "IMAQ AVI Close"("Avi Refnum"=w3370) -> ()  [unwired: 1 in, 10 out]
              }
            }
            n2271 = local write "Video Index"(w3369) -> ()
            n2272 = call "IMAQ AVI Create"("Frames Per Second"=u32 30, "AVI Path"=w3359) -> ("Avi Refnum"=w3367:T36)  [unwired: 5 in, 4 out]
          }
        }
        n2273 = Equal To 0?(x=w3350) -> (x = 0?=w3349:bool)
        n2274 = Select(t=w3340, s=w3341, f=w3338) -> (s? t:f=w3339:T36)
        n2275 = feedback-in #1(w3339) -> ()
        n2276 = case shown="True" w3349 {
          tunnel: w3348 -> [w3371 w3405]
          tunnel: w3347 -> [_ w3404]
          tunnel: [w3371 w3401] -> w3345
          tunnel: w3344 -> [_ w3386]
          tunnel: w3333 -> [_ w3390]
          tunnel: w3339 -> [_ w3388]
          tunnel: w3331 -> [_ w3383]
          tunnel: w3330 -> [_ w3382]
          frame False {
          }
          frame True {
            w3395 = u32 0 ("X-offset IN")
            n2277 = call "DMR_GetImageRequestBufferData.vi"("driver handle IN"=w3405, "request number IN"=w3404) -> ("width OUT"=w3394:i32, "height OUT"=w3393:i32, "driver handle OUT"=w3400:i32, "request number OUT"=w3399:i32, "bytes per pixel OUT"=w3396:i32)  [unwired: 13 out]
            n2278 = call "DMR_GetImageRequestBufferImageData.vi"("driver handle IN"=w3400, "request number IN"=w3399, "bytes per pixel IN"=w3396, "X-offset IN"=w3395, "Y-offset IN"=w3395, "height IN"=w3393, "width IN"=w3394) -> ("driver handle OUT"=w3398:u32, "request number OUT"=w3397:u32, "image OUT"=w3375:u32[][])  [unwired: 10 out]
            n2279 = Transpose 2D Array(2D array=w3375) -> (transposed array=w3381:u32[][])
            n2280 = Select(t=w3381, s="Flip Y (or X)", f=w3375) -> (s? t:f=w3380:u32[][])
            n2281 = call "DMR_ImageRequestUnlock.vi"("request number IN"=w3397, "driver handle IN"=w3398) -> ("driver handle OUT"=w3403:i32)  [unwired: 1 in, 2 out]
            n2282 = for {
              tunnel: w3380 -> [w3440] mode=indexing
              tunnel: [w3439] -> w3378 mode=indexing
              n2283 = Reverse 1D Array(array=w3440) -> (reversed array=w3439:u32[])
            }
            n2284 = call "DMR_ImageRequestSingle.vi"("request control IN"=0, "driver handle IN"=w3403) -> ("driver handle OUT"=w3401:i32)  [unwired: 3 out]
            n2285 = Transpose 2D Array(2D array=w3378) -> (transposed array=w3379:u32[][])
            n2286 = Select(t=w3379, s="Flip Y (or X)", f=w3378) -> (s? t:f=w3376:u32[][])
            n2287 = Select(t=w3376, s="Flip Image", f=w3375) -> (s? t:f=w3373:u32[][])
            n2288 = case shown="True" "Averaging" {
              tunnel: w3373 -> [w3443 w3448]
              tunnel: [w3443 w3447] -> w3387
              tunnel: w3390 -> [_ w3445]
              frame False {
              }
              frame True {
                (unwired) 1
                w3453 = 1
                n2289 = feedback #2(w3445) -> (w3444:u32[][])
                n2290 = Add(x=w3448, y=w3444) -> (x+y=w3449:u32[][])
                n2291 = Select(t=w3445, s="Reset Averaging", f=w3449) -> (s? t:f=w3451:u32[][])
                n2292 = feedback-in #2(w3451) -> ()
                n2293 = feedback #3(w3453) -> (w3446:i32)
                n2294 = Divide(x=w3449, y=w3446) -> (x/y=w3450:dbl[][])
                n2295 = Increment(x=w3446) -> (x+1=w3454:i32)
                n2296 = To Unsigned Long Integer(number=w3450) -> (unsigned 32bit integer=w3447:u32[][])
                n2297 = Select(t=w3453, s="Reset Averaging", f=w3454) -> (s? t:f=w3452:i32)
                n2298 = feedback-in #3(w3452) -> ()
              }
            }
            n2299 = case shown="True" "Zoom video window" {
              tunnel: w3387 -> [_ w3419]
              tunnel: w3383 -> [_ w3418]
              frame False {
              }
              frame True {
                n2300 = To Double Precision Float(number=w3419) -> (double precision float=w3416:dbl[][])
                n2301 = In Range and Coerce(upper limit="Intensity Upper", x=w3416, lower limit="Intensity Lower") -> (coerced(x)=w3415:dbl[][])  [unwired: 1 out]
                n2302 = Subtract(x="Intensity Upper", y="Intensity Lower") -> (x-y=w3412:dbl)
                n2303 = Subtract(x=w3415, y="Intensity Lower") -> (x-y=w3413:dbl[][])
                n2304 = Divide(x=w3413, y=w3412) -> (x/y=w3414:dbl[][])
                n2305 = Multiply(x=255.0, y=w3414) -> (x*y=w3410:dbl[][])
                n2306 = To Unsigned Byte Integer(number=w3410) -> (unsigned 8bit integer=w3417:u8[][])
                n2307 = call "IMAQ ArrayToImage"("Image Pixels (U8)"=w3417, "Image"=w3418) -> ("Image Out"=w3406:T2)  [unwired: 4 in, 5 out]
                n2308 = First Call?() -> (First Call?: T/F=w3407:bool)
                n2309 = case shown="True" w3407 {
                  tunnel: w3406 -> [w3420 w3431]
                  frame False {
                    n2310 = flat-sequence {
                      tunnel: w3420 -> [w3426]
                      frame #0 {
                        w3423 = FALSE ("Get/Set Status? (Set)")
                        w3422 = 0 ("Window Number (0...15)")
                        n2311 = call "IMAQ WindSize"("Get/Set Status? (Set)"=w3423, "Window Number"=w3422) -> ("Width & Height out"=→"Window Size":cluster{"Width":i32, "Height":i32})  [unwired: 4 in, 2 out]
                        n2312 = call "IMAQ WindMove"("Window Number (0...15)"=w3422, "Get/Set Status? (Set)"=w3423) -> ("Coordinates (screen)"=→"Window Position":cluster{"X Position":i32, "Y Position":i32})  [unwired: 3 in, 1 out]
                        n2313 = call "IMAQ WindDraw"("Resize to Image Size? (Y)"=FALSE, "Window Number (0...15)"=w3422, "Image"=w3426) -> ()  [unwired: 7 in, 2 out]
                      }
                      frame #1 {
                        n2314 = call "IMAQ WindZoom 2"("Center Point"="Center Point", "Zoom to Fit? (False)"=FALSE, "Zoom Factor"="Zoom Factor") -> ()  [unwired: 5 in, 4 out]
                      }
                    }
                  }
                  frame True {
                    n2315 = flat-sequence {
                      tunnel: w3431 -> [w3434]
                      tunnel: [w3432] -> w3430
                      tunnel: w3430 -> [w3436]
                      frame #0 {
                        w3433 = TRUE ("Resize to Image Size? (Y)")
                        w3432 = 0 ("Window Number (0...15)")
                        n2316 = call "IMAQ WindNonTearing"("Window Number"=w3432, "NonTearing? (True)"=w3433) -> ()  [unwired: 8 in, 2 out]
                        n2317 = call "IMAQ WindDraw"("Resize to Image Size? (Y)"=w3433, "Window Number (0...15)"=w3432, "Image"=w3434) -> ()  [unwired: 7 in, 2 out]
                      }
                      frame #1 {
                        n2318 = call "IMAQ WindSize"("Scrollbars? (N)"=FALSE, "Width & Height"="Initial Window Size", "Window Number"=w3436) -> ()  [unwired: 3 in, 3 out]
                        n2319 = call "IMAQ WindMove"("Window Number (0...15)"=w3436, "Coordinates (screen)"="Initial Window Position") -> ()  [unwired: 3 in, 2 out]
                      }
                    }
                  }
                }
              }
            }
            n2320 = To Unsigned Byte Integer(number=w3387) -> (unsigned 8bit integer=w3385:u8[][])
            n2321 = call "IMAQ ArrayToImage"("Image Pixels (U8)"=w3385, "Image"=w3386) -> ("Image Out"=w3384:T2)  [unwired: 4 in, 5 out]
            "Primary Video Display" <- w3384
            n2322 = case shown="True" "Save Video" {
              tunnel: w3388 -> [_ w3442]
              tunnel: w3384 -> [_ w3441]
              frame False {
              }
              frame True {
                n2323 = call "IMAQ AVI Write Frame"("Image"=w3441, "Avi Refnum"=w3442) -> ()  [unwired: 2 in, 8 out]
              }
            }
            n2324 = case shown="True" "Save Image" {
              tunnel: w3385 -> [_ w3457]
              tunnel: w3382 -> [_ w3456]
              frame False {
              }
              frame True {
                n2325 = call <vilib>:"Flatten Pixmap.vi"("colors"=w3456, "8-bit pixmap"=w3457) -> ("image data"=w3463:T37)  [unwired: 4 in, 5 out]
                n2326 = call "Create new save file.vi"("Insert"="video_frame_" ("string"), "Ext"=".bmp" ("string"), "Index In"="Image Index") -> ("Path Out"=w3459:path, "Index Out"=w3464:dbl)
                n2327 = Increment(x=w3464) -> (x+1=w3458:dbl)
                n2328 = local write "Image Index"(w3458) -> ()
                n2329 = call <vilib>:"Write BMP File.vi"("image data"=w3463, "path to BMP file"=w3459) -> ()  [unwired: 1 in, 9 out]
              }
            }
          }
        }
        n2330 = node-c288(w3334) -> ()  [unwired: 1 out]
      }
      n2331 = node-c288(w3318) -> ()  [unwired: 1 out]
      n2332 = call "DMR_CloseDevice.vi"("driver handle IN"=w3323) -> ()  [unwired: 1 in, 4 out]
    }
    frame #4 {
      n2333 = call "DMR_Close.vi"() -> ()  [unwired: 1 out]
    }
  }
  n2334 = node-c288(i64 1 ("Period"), 1 ("Processor")) -> (w206:T23)  [unwired: 2 out]
  n2335 = timed-loop "Main data acquisition loop (get data, process data for display, and save data to disk)" {
    tunnel: w23 -> [w3778]
    tunnel: w94 -> [w3777]
    tunnel: [w3807] -> w298
    tunnel: [w3802] -> w296
    timing: w206 -> [_]
    timing-out: [_] -> w205
    tunnel: w111 -> [w3631]
    stop <- "Stop All" stop-if-true
    w3548 = "Initialize"
    # "Fluorescence data into FIFO for external control vi's\n(e.g., fluorescence triggering) - Duncan Nall"
    n2336 = node-c288() -> ()  [unwired: 2 out]
    n2337 = First Call?() -> (First Call?: T/F=w3583:bool)
    n2338 = Or(x="Reset", y=w3583) -> (x .or. y?=w3584:bool)
    n2339 = local read "Flushing P1"() -> (w3503:bool)
    n2340 = case "Reset data stream (manual reset or at begining of some rastering and imaging)" shown="True" w3584 {
      tunnel: w3778 -> [w4848 w4856]
      tunnel: w3777 -> [w4847 w4855]
      tunnel: [w4848 w4850] -> w3773
      tunnel: [w4847 w4849] -> w3772
      frame False {
      }
      frame True {
        w4853 = TRUE ("AI to FIFO")
        n2341 = local write "Overflow (data lost)"(FALSE ("Overflow (data lost)")) -> ()
        n2342 = call "reset FPGA DMA.vi"("error in"=w4855, "FPGA VI Reference In"=w4856) -> ("error out"=w4851:errorcluster, "FPGA VI Reference Out"=w4852:T20)
        n2343 = xnode "Read/Write Control"("FPGA VI Reference In"=w4852, "error in"=w4851, "AI to FIFO"=w4853, "APD to FIFO"=w4853) -> ("FPGA VI Reference Out"=w4850:T20, "error out"=w4849:errorcluster)
      }
    }
    n2344 = case shown="True" w3503 {
      frame False {
      }
      frame True {
        n2345 = local read "Flush rate (uL/m) P1"() -> (w3837:dbl)
        n2346 = local read "HP1 Flush Time (s)"() -> (w3846:dbl)
        n2347 = local read "DMA Update Period (s)"() -> (w3840:dbl)
        n2348 = Divide(x=w3837, y=60.0) -> (x/y=w3838:dbl)
        n2349 = Divide(x=w3846, y=w3840) -> (x/y=w3835:dbl)
        n2350 = feedback #4(0) -> (w3844:i32)
        n2351 = Increment(x=w3844) -> (x+1=w3834:i32)
        n2352 = Greater?(x=w3834, y=w3835) -> (0:w3843:bool)
        n2353 = Compound Arithmetic op=MULTIPLY(w3840, w3834, w3838) -> (→"P1 Flush Volume (uL)":dbl)
        n2354 = Divide(x=w3834, y=w3835) -> (x/y=→"P1 Flushing Bar":dbl)
        n2355 = case shown="True" w3843 {
          tunnel: w3834 -> [w3847 _]
          tunnel: [w3847 0] -> w3842
          frame False {
          }
          frame True {
            w3848 = FALSE ("Flushing P1")
            n2356 = local write "Inject Pump 1"(w3848) -> ()
            n2357 = local write "Flushing P1"(w3848) -> ()
            n2358 = property on="Clear Volume P1" class="Bool (strict)"("Val(Sgnl)"=TRUE ("Value (Signaling)")) -> ()  [unwired: 2 in, 2 out]
          }
        }
        n2359 = feedback-in #4(w3842) -> ()
      }
    }
    n2360 = Or(x="Start AOD Scan", y="Trap Raster Scan") -> (x .or. y?=w3729:bool)
    n2361 = case "Start AOM raster scan" shown="True" w3729 {
      tunnel: w3773 -> [w4698 w4708]
      tunnel: w3772 -> [w4697 w4707]
      tunnel: [w4698 w4701] -> w3771
      tunnel: [w4697 w4700] -> w3770
      frame False {
      }
      frame True {
        n2362 = case shown="True" "Restart DMA? (AOD)" {
          tunnel: [w4746 w4748] -> w4702
          tunnel: [w4745 w4747] -> w4703
          tunnel: w4708 -> [w4746 w4750]
          tunnel: w4707 -> [w4745 w4749]
          frame False {
          }
          frame True {
            n2363 = local write "Overflow (data lost)"(FALSE ("Overflow (data lost)")) -> ()
            n2364 = call "reset FPGA DMA.vi"("error in"=w4749, "FPGA VI Reference In"=w4750) -> ("error out"=w4747:errorcluster, "FPGA VI Reference Out"=w4748:T20)
          }
        }
        n2365 = local write "Trap Raster Scan"(FALSE ("Trap Raster Scan")) -> ()
        n2366 = case shown="True" "Move MCL Also?" {
          tunnel: w4703 -> [w4711 w4740]
          tunnel: w4702 -> [w4712 w4741]
          tunnel: [w4710 w4744] -> w4701
          tunnel: [w4709 w4743] -> w4700
          frame False {
            w4713 = TRUE ("AI to FIFO")
            n2367 = xnode "Read/Write Control"("FPGA VI Reference In"=w4712, "error in"=w4711, "AI to FIFO"=w4713, "APD to FIFO"=w4713, "Start scan"=w4713) -> ("FPGA VI Reference Out"=w4710:T20, "error out"=w4709:errorcluster)
          }
          frame True {
            w4737 = FALSE ("1D or 2D Scan?")
            w4742 = TRUE ("AI to FIFO")
            # "Count for MCL loop"
            # "N total cycles"
            # "N steps"
            # "V_int"
            n2368 = local read "Scan Range (nm)"() -> (w4719:dbl)
            n2369 = local read "Number of F/B Scans (AOD)"() -> (w4736:u16)
            n2370 = Sign(1:w4719) -> (0:w4718:dbl)
            n2371 = Compound Arithmetic op=MULTIPLY(w4719, "MCL Step Position Ratio", "MCL/AOM Scale Tweak") -> (w4723:dbl)
            n2372 = Negate(x=w4718) -> (-x=w4715:dbl)
            n2373 = Multiply(x=w4715, y="MCL Step Increment (V_int)") -> (x*y=w4717:dbl)
            n2374 = Divide(x=w4723, y="MCL X Cal (nm/V)") -> (x/y=w4729:dbl)
            n2375 = Multiply(x=32767.0 ("y"), y=w4729) -> (x*y=w4735:dbl)
            n2376 = local read "Total Counts (ticks)"() -> (w4720:u16)
            n2377 = local read "Cycles/step (AOD)"() -> (w4731:u64)
            n2378 = local read "Scan steps (AOD)"() -> (w4732:u64)
            n2379 = Divide(x=w4735, y=10.0) -> (x/y=w4728:dbl)
            n2380 = Divide(x=w4728, y="MCL Step Increment (V_int)") -> (x/y=w4726:dbl)
            n2381 = Absolute Value(x=w4726) -> (abs(x)=w4714:dbl)
            n2382 = Compound Arithmetic op=MULTIPLY(w4732, w4731, w4720) -> (w4727:u64)
            n2383 = local write "wait to reset values"(w4742) -> ()
            n2384 = local write "MCL Scanning"(w4742) -> ()
            n2385 = Divide(x=w4727, y=w4714) -> (x/y=w4724:dbl)
            "MCL Count" <- w4724
            n2386 = xnode "Read/Write Control"("FPGA VI Reference In"=w4741, "error in"=w4740, "Scan steps (MCL)"=w4714, "Number of scans (MCL)"=w4736, "Cycles per step (MCL)"=u64 1, "Scan freq.  increment (MCL)"=w4717, "1D or 2D Scan?"=w4737, "MCL Scan Axis"=w4737, "Cont. Scan (MCL)"=w4737, "MCL count"=w4724) -> ("FPGA VI Reference Out"=w4739:T20, "error out"=w4738:errorcluster)
            n2387 = xnode "Read/Write Control"("FPGA VI Reference In"=w4739, "error in"=w4738, "AI to FIFO"=w4742, "APD to FIFO"=w4742, "Start scan"=w4742, "Start scan (MCL)"=w4742) -> ("FPGA VI Reference Out"=w4744:T20, "error out"=w4743:errorcluster)
          }
        }
        "Raster Scanning..." <- TRUE ("Scanning...")
      }
    }
    n2388 = local read "Flushing P3"() -> (w3504:bool)
    n2389 = case "Keep track of when Harvard Pump 3 is done flushing" shown="True" w3504 {
      frame False {
      }
      frame True {
        n2390 = local read "Flush rate (uL/m) P3"() -> (w3854:dbl)
        n2391 = local read "DMA Update Period (s)"() -> (w3856:dbl)
        n2392 = local read "HP3 Flush Time (s)"() -> (w3863:dbl)
        n2393 = Divide(x=w3854, y=60.0) -> (x/y=w3852:dbl)
        n2394 = feedback #5(0) -> (w3861:i32)
        n2395 = Increment(x=w3861) -> (x+1=w3855:i32)
        n2396 = Divide(x=w3863, y=w3856) -> (x/y=w3857:dbl)
        n2397 = Greater?(x=w3855, y=w3857) -> (0:w3860:bool)
        n2398 = Compound Arithmetic op=MULTIPLY(w3856, w3855, w3852) -> (→"P3 Flush Volume (uL)":dbl)
        n2399 = case shown="True" w3860 {
          tunnel: w3855 -> [w3864 _]
          tunnel: [w3864 0] -> w3859
          frame False {
          }
          frame True {
            w3865 = FALSE ("Flushing P3")
            n2400 = local write "Inject Pump 3"(w3865) -> ()
            n2401 = local write "Flushing P3"(w3865) -> ()
            n2402 = property on="Clear Volume P3" class="Bool (strict)"("Val(Sgnl)"=TRUE ("Value (Signaling)")) -> ()  [unwired: 2 in, 2 out]
          }
        }
        n2403 = feedback-in #5(w3859) -> ()
        n2404 = Divide(x=w3855, y=w3857) -> (x/y=→"P3 Flushing Bar":dbl)
      }
    }
    n2405 = And(x="Save scans", y=w3729) -> (x .and. y?=w3769:bool)
    n2406 = Compound Arithmetic op=OR("Start MCL Scan", "Confocal Image", "Confocal Linescan") -> (w3727:bool)
    n2407 = And(x="Save Data (MCL)", y=w3727) -> (x .and. y?=w3768:bool)
    n2408 = case "Start MCL raster scan" shown="True" w3727 {
      tunnel: w3771 -> [w4310 w4326]
      tunnel: w3770 -> [w4309 w4325]
      tunnel: [w4310 w4321] -> w3630
      tunnel: [w4309 w4320] -> w3629
      tunnel: [FALSE w4319] -> w3754
      tunnel: "Start MCL Scan" -> [_ w4314]
      tunnel: "Confocal Image" -> [_ w4313]
      tunnel: "Confocal Linescan" -> [_ _]
      frame False {
      }
      frame True {
        w4319 = TRUE
        n2409 = case shown="True" "Restart DMA? (MCL)" {
          tunnel: [w4371 w4373] -> w4324
          tunnel: [w4370 w4372] -> w4323
          tunnel: w4326 -> [w4371 w4376]
          tunnel: w4325 -> [w4370 w4375]
          frame False {
          }
          frame True {
            n2410 = call "reset FPGA DMA.vi"("error in"=w4375, "FPGA VI Reference In"=w4376) -> ("error out"=w4372:errorcluster, "FPGA VI Reference Out"=w4373:T20)
            n2411 = local write "Overflow (data lost)"(FALSE ("Overflow (data lost)")) -> ()
          }
        }
        n2412 = case shown="False" w4314 {
          selector: w4314 -> [_ w4330]
          tunnel: w4313 -> [w4329 _]
          tunnel: [w4329 w4330] -> w4312
          frame False {
            n2413 = property on="2D or 1D Scan" class="Bool (strict)"("Val(Sgnl)"=w4329) -> ()  [unwired: 2 in, 2 out]
            n2414 = property on="Confocal Image" class="Bool (strict)"("Value"=FALSE ("Start Confocal Map")) -> ()  [unwired: 2 in, 2 out]
          }
          frame True {
          }
        }
        n2415 = local write "MCL Scanning"(w4319) -> ()
        n2416 = local read "AO1"() -> (w4316:dbl)
        n2417 = local read "AO2"() -> (w4315:dbl)
        n2418 = case shown="True" "Center Scan" {
          tunnel: w4324 -> [w4337 w4369]
          tunnel: w4323 -> [w4336 w4368]
          tunnel: [w4335 w4367] -> w4321
          tunnel: [w4334 w4366] -> w4320
          tunnel: [w4332 w4353] -> w4318
          tunnel: [w4331 w4352] -> w4317
          tunnel: w4316 -> [w4332 w4358]
          tunnel: w4315 -> [w4331 w4361]
          tunnel: w4312 -> [_ _]
          frame False {
            w4333 = TRUE ("AI to FIFO")
            n2419 = xnode "Read/Write Control"("FPGA VI Reference In"=w4337, "error in"=w4336, "AI to FIFO"=w4333, "APD to FIFO"=w4333, "Start scan (MCL)"=w4333) -> ("FPGA VI Reference Out"=w4335:T20, "error out"=w4334:errorcluster)